vi "UHR-Fleezers Control (host) - 12.8.vi"() -> ()   [LabVIEW 2012] (continued)
  T33 = cluster{"Left":i32, "Top":i32, "Width":u32, "Height":u32}
  T34 = cluster{cluster{"Left":i32, "Top":i32, "Width":u32, "Height":u32}}[]
  T35 = enum32{"setting", "request", "request control", "info", "statistics", "system settings", "I/O sub system", "HRT control", "camera descriptions", "device specific data", "event sub system settings", "event sub system results", "image memory manager"}
  T36 = typedef "IMAQ AVI2 Refnum.ctl" = refnum<k20>
  T37 = typedef "imagedata.ctl" = cluster{"image type":i32, "image depth":i32, "image":u8[], "mask":u8[], "colors":u32[], "Rectangle":cluster{"left":i16, "top":i16, "right":i16, "bottom":i16}}
  T38 = enum32{"Normal Display", "Dual Display (APD)", "FFT", "High Res Display"}
  T39 = cluster{"Origin Pixel":cluster{"X":sgl, "Y":sgl}, "Angle Relative to Horizontal (deg)":sgl, "Axis Reference":u32}
  T40 = typedef "Simple Grid Descriptor" = cluster{"X Step":sgl, "Y Step":sgl, "Unit":T41}
  T41 = typedef "Image Unit" = enum32{"Undefined", "Angström", "Micrometer", "Millimeter", "Centimeter", "Meter", "Kilometer", "Microinch", "Inch", "Feet", "Nautical miles", "Standard miles", "Steps"}
  T42 = cluster{"averaging mode":u16, "weighting mode":u16, "number of averages":u32}
  T43 = cluster{"dB On (F)":bool, "unwrap phase (F)":bool, "convert to degree (F)":bool}
  T44 = cluster{string, string, string, string, string, string, string, string}
  T45 = cluster{string, string, string, string, string, string, string, string, string, string, string, string}
  T46 = cluster{string, string, string, string, string, string, string, string, string, string, string, string, string}
  T47 = cluster{string, string, string, string, string, string, string, string, string, string, string, string, string, string}
  T48 = cluster{"BD 1 Frequency 1 (MHz)":dbl, "BD 1 Frequency 2 (MHz)":dbl}
  T49 = cluster{"f0":dbl, "df":dbl, "magnitude":dbl[]}[][]
  T50 = cluster{"Comment (data description)":string, "Channel 1 Buffer":string, "Channel 2 Buffer":string, "Channel 3 Buffer":string, "Title":string, "DNA Construct":string, "Bead diameter":dbl, "Name":string}
diagram:
  w18 = u16 10 items=["1.0"=10, "1.5"=15, "2.0"=20] ("stop bits (10: 1 bit)")
  w34 = u16 20 items=["1.0"=10, "1.5"=15, "2.0"=20] ("stop bits (10: 1 bit)")
  w37 = u16 20 items=["1.0"=10, "1.5"=15, "2.0"=20] ("stop bits (10: 1 bit)")
  w45 = u16 20 items=["1.0"=10, "1.5"=15, "2.0"=20] ("stop bits (10: 1 bit)")
  w24 = T19 2 items=["Grayscale (U8)", "Grayscale (I16)", "Grayscale (SGL)", "Complex (CSG)", "RGB (U32)", "HSL (U32)", "RGB (U64)", "Grayscale (U16)"] ("Image Type")
  # "Settings to help prevent AOM/D damage"
  # "Initialize the FPGA DAQ card itself"
  # "Reset the DAQ card."
  # "Specify the DAQ card and the FPGA code to run"
  # "Bottom 1 Harvard"
  # "Top 3 Harvard"
  # "Center Harvard"
  # "Bottom 1 Harvard"
  # "Top 3 Harvard"
  # "Center Harvard"
  n1 = case "Trap X limits" shown="\"AOD3Sets\"" "1axis AOM vs 2 axis AOD" {
    tunnel: [T16 {"Minimum"=0.0, "Maximum"=40.0, "Increment"=0.1} ("Min Max Inc") T16 {"Minimum"=0.0, "Maximum"=40.0, "Increment"=0.1} ("Min Max Inc") T16 {"Minimum"=60.0, "Maximum"=90.0, "Increment"=1.0} ("Min Max Inc")] -> w9
    tunnel: [T16 {"Minimum"=0.0, "Maximum"=45.0, "Increment"=1.0} ("Data Entry Limits") T16 {"Minimum"=0.0, "Maximum"=45.0, "Increment"=1.0} ("Data Entry Limits") T16 {"Minimum"=0.0, "Maximum"=50.0, "Increment"=1.0} ("Data Entry Limits")] -> w7
    frame "2axisAOD" {
      w81 = u16 300 ("DIO count 1 (ticks)")
      # "Amp Limits"
      # "Freq Limits"
      n2 = disable-structure shown="Disabled" {
        frame Disabled {
          w87 = 35.0 ("BD 1 Amplitude 1 (%)")
          w88 = 30.0 ("BD 1 Frequency 1 (MHz)")
          n3 = local write "BD 1 Frequency 1 (MHz)"(w88) -> ()
          n4 = local write "BD 1 Frequency 2 (MHz)"(w88) -> ()
          n5 = local write "BD 1 Amplitude 2 (%)"(w87) -> ()
          n6 = local write "BD 1 Amplitude 1 (%)"(w87) -> ()
          n7 = local write "BD 2 Frequency 1 (MHz)"(w88) -> ()
          n8 = local write "BD 2 Amplitude 1 (%)"(w87) -> ()
          n9 = local write "BD 2 Frequency 2 (MHz)"(w88) -> ()
          n10 = local write "BD 2 Amplitude 2 (%)"(w87) -> ()
        }
        frame Enabled {
        }
      }
      n11 = local write "All FB On/Off"(FALSE ("All FB On/Off")) -> ()
      n12 = local write "BD 2 Delay (Ticks)"(u8 108 ("BD 2 Delay (Ticks)")) -> ()
      n13 = local write "Number Interlace Sets"(u8 2 ("Number Interlace Sets")) -> ()
      n14 = local write "DIO count 2 (ticks)"(w81) -> ()
      n15 = local write "DIO count 1 (ticks)"(w81) -> ()
    }
    frame "AOD3Sets" {
      w89 = u16 200 ("DIO count 1 (ticks)")
      # "Amp Limits"
      # "Freq Limits"
      n16 = disable-structure shown="Disabled" {
        frame Disabled {
          w95 = 35.0 ("BD 1 Amplitude 1 (%)")
          w96 = 30.0 ("BD 1 Frequency 1 (MHz)")
          n17 = local write "BD 1 Frequency 1 (MHz)"(w96) -> ()
          n18 = local write "BD 1 Frequency 2 (MHz)"(w96) -> ()
          n19 = local write "BD 1 Amplitude 2 (%)"(w95) -> ()
          n20 = local write "BD 1 Amplitude 1 (%)"(w95) -> ()
          n21 = local write "BD 2 Frequency 1 (MHz)"(w96) -> ()
          n22 = local write "BD 2 Amplitude 1 (%)"(w95) -> ()
          n23 = local write "BD 2 Frequency 2 (MHz)"(w96) -> ()
          n24 = local write "BD 2 Amplitude 2 (%)"(w95) -> ()
        }
        frame Enabled {
        }
      }
      n25 = local write "All FB On/Off"(FALSE ("All FB On/Off")) -> ()
      n26 = local write "BD 2 Delay (Ticks)"(u8 0 ("BD 2 Delay (Ticks)")) -> ()
      n27 = local write "Number Interlace Sets"(u8 3 ("Number Interlace Sets")) -> ()
      n28 = local write "DIO count 2 (ticks)"(w89) -> ()
      n29 = local write "DIO count 1 (ticks)"(w89) -> ()
    }
    frame "1axis", Default {
      # "Amp Lmits"
      # "Freq Limits"
    }
  }
  n30 = xnode "Open FPGA VI Reference"("resource name"=T18 "750kHzDAQ") -> ("FPGA VI Reference Out"=w14:T20, "error out"=w13:errorcluster)  [unwired: 1 in]
  n31 = xnode "Invoke Method"("FPGA VI Reference In"=w14, "error in"=w13) -> ("FPGA VI Reference Out"=w6:T20, "error out"=→"FPGA error out":errorcluster)
  n32 = flat-sequence "Safety limits on RF frequencies and amplitudes (for AOM protection)" {
    tunnel: [w101] -> w1
    tunnel: [w100] -> w3
    tunnel: [w102] -> w4
    tunnel: [w103] -> w2
    tunnel: w9 -> [w101]
    tunnel: w7 -> [w100]
    tunnel: w6 -> [w99]
    tunnel: [w99] -> w5
    frame #0 {
      w103 = T16 {"Minimum"=0.0, "Maximum"=40.0, "Increment"=0.1} ("Min Max Inc")
      w102 = T16 {"Minimum"=0.0, "Maximum"=45.0, "Increment"=1.0} ("Data Entry Limits")
      n33 = property on="BD 2 Frequency 1 (MHz)" class="DigNum (strict)"("Data Range"=w103) -> ()  [unwired: 2 in, 2 out]
      n34 = property on="BD 2 Frequency 3 (MHz)" class="DigNum (strict)"("Data Range"=w103) -> ()  [unwired: 2 in, 2 out]
      n35 = property on="BD 2 Frequency 2 (MHz)" class="DigNum (strict)"("Data Range"=w103) -> ()  [unwired: 2 in, 2 out]
      n36 = property on="BD 1 Frequency 1 (MHz)" class="DigNum (strict)"("Data Range"=w101) -> ()  [unwired: 2 in, 2 out]
      n37 = property on="BD 1 Frequency 2 (MHz)" class="DigNum (strict)"("Data Range"=w101) -> ()  [unwired: 2 in, 2 out]
      n38 = property on="BD 1 Frequency 3 (MHz)" class="DigNum (strict)"("Data Range"=w101) -> ()  [unwired: 2 in, 2 out]
      n39 = property on="BD 2 Amplitude 1 (%)" class="DigNum (strict)"("Data Range"=w102) -> ()  [unwired: 2 in, 2 out]
      n40 = property on="BD 2 Amplitude 2 (%)" class="DigNum (strict)"("Data Range"=w102) -> ()  [unwired: 2 in, 2 out]
      n41 = property on="BD 2 Amplitude 3 (%)" class="DigNum (strict)"("Data Range"=w102) -> ()  [unwired: 2 in, 2 out]
      n42 = property on="BD 1 Amplitude 3 (%)" class="DigNum (strict)"("Data Range"=w100) -> ()  [unwired: 2 in, 2 out]
      n43 = property on="BD 1 Amplitude 2 (%)" class="DigNum (strict)"("Data Range"=w100) -> ()  [unwired: 2 in, 2 out]
      n44 = property on="BD 1 Amplitude 1 (%)" class="DigNum (strict)"("Data Range"=w100) -> ()  [unwired: 2 in, 2 out]
      "X RF Frequency Limits (MHz)" <- w101
      "X RF Amplitude Limits (%)" <- w100
      "Y RF Amplitude Limits (%)" <- w102
      "Y RF Frequency Limits (MHz)" <- w103
    }
  }
  n45 = stacked-sequence "Host initialization sequence - order matters!" {
    tunnel: w5 -> [_ w106 w204 _ w271 w279 w325 w350 w380]
    tunnel: [_ _ _ _ _ _ _ _ w380] -> w11
    tunnel: [_ _ _ _ _ _ _ _ w379] -> w10
    tunnel: w4 -> [_ _ _ _ _ _ w322 _ _]
    tunnel: w3 -> [_ _ _ _ _ _ w321 _ _]
    tunnel: w2 -> [_ _ _ _ _ _ w320 _ _]
    tunnel: w1 -> [_ _ _ _ _ _ w319 _ _]
    frame #0 {
    }
    frame #1 {
      w139 = 10.0 ("y")
      w140 = 32767.0 ("y")
      w124 = 6.0  # clock mult.
      w123 = 49152000.0  # TCXO frequ.
      # "Initialize some FPGA settings"
      n46 = Build Array("DIO count 1 (ticks)", "DIO count 2 (ticks)", "DIO count 3 (ticks)") -> (w174:u16[])
      n47 = local read "AO1"() -> (w145:dbl)
      n48 = local read "AO2"() -> (w146:dbl)
      n49 = local read "Scan Increment (MHz)"() -> (w128:dbl)
      n50 = property on="AI Count (ticks)" class="DigNum (strict)"("Val(Sgnl)"="AI Count (ticks)") -> ()  [unwired: 2 in, 2 out]
      n51 = local read "Continuous MCL Scanning"() -> (w158:bool)
      n52 = local read "Fast Scan Dir"() -> (w159:bool)
      n53 = local read "Number of scans (MCL)"() -> (w157:u64)
      n54 = Multiply(x=w145, y=w140) -> (x*y=w143:dbl)
      n55 = Multiply(x=w146, y=w140) -> (x*y=w141:dbl)
      n56 = Divide(x=40000000.0, y="AI Count (ticks)") -> (x/y=w163:dbl)
      n57 = Divide(x=w143, y=w139) -> (x/y=w144:dbl)
      n58 = Divide(x=w141, y=w139) -> (x/y=w142:dbl)
      n59 = To Word Integer(number=w144) -> (16bit integer=w147:i16)
      n60 = To Word Integer(number=w142) -> (16bit integer=w148:i16)
      n61 = Not(x=w159) -> (.not. x?=w160:bool)
      n62 = local read "Cycles/step (MCL)"() -> (w156:u64)
      n63 = Multiply(x=w128, y=1000.0) -> (x*y=w121:dbl)
      n64 = local read "Scan steps (MCL)"() -> (w155:u64)
      n65 = local write "Trap Pos FIFO Timeout"(u16 0 ("Trap Pos FIFO Timeout")) -> ()
      n66 = local read "Desired Scan Incr (V)"() -> (w153:dbl)
      n67 = local write "AI rate (Hz)"(w163) -> ()
      n68 = Scale By Power Of 2(n=48, x=w121) -> (x*2^n=w120:dbl)
      n69 = Unbundle By Name(cluster{"output high":i16, "output low":i16} {"output high"=3000, "output low"=0} ("FB output range 1")) -> ("output high"=w193:i16, "output low"=w194:i16)
      n70 = Multiply(x=w123, y=w124) -> (x*y=w125:dbl)
      n71 = Divide(x=w120, y=w125) -> (x/y=w126:dbl)
      n72 = local read "Setpoints (V)"() -> (w113:cluster{"Set 1":dbl, "Set 2":dbl})
      n73 = To Quad Integer(1:w126) -> (0:w129:i64)
      n74 = Multiply(x=w153, y=32767.0) -> (x*y=w151:dbl)
      n75 = Divide(x=w163, y="FPGA Ave.") -> (x/y=w162:dbl)
      n76 = local read "Trap Intensity PID Gains"() -> (w118:T9)
      n77 = local read "Next trap write delay (ticks)"() -> (w197:u8)
      n78 = local read "XY phase ext loop method"() -> (w198:bool)
      n79 = local read "Amp switch delay 2"() -> (w199:u8)
      n80 = local read "BD 2 Delay (Ticks) 2"() -> (w200:u8)
      n81 = local read "BD 1 Delay (ticks) 2"() -> (w201:u8)
      n82 = local write "Ave. Rate (Hz)"(w162) -> ()
      n83 = Reciprocal(x=w162) -> (1/x=w161:dbl)
      n84 = local read "Number Interlace Sets"() -> (w181:u8)
      n85 = Split 1D Array(array=w174, index=w181) -> (first subarray=w172:u16[])  [unwired: 1 out]
      n86 = Add Array Elements(numeric array=w172) -> (sum=w173:u16)
      n87 = local write "Ave. Period (s)"(w161) -> ()
      n88 = local read "# Samples/channel"() -> (w136:u32)
      n89 = local read "Number of F/B Scans (AOD)"() -> (w135:u16)
      n90 = local read "Not-Interlacing Set"() -> (w182:enum32{"Set 1", "Set 2", "Set 3"})
      n91 = To Unsigned Byte Integer(number=w182) -> (unsigned 8bit integer=w176:u8)
      n92 = Index Array(array=w174, index=w176) -> (element=w175:u16)
      n93 = local read "Feedback On/Off"() -> (w110:cluster{"Set 1":bool, "Set 2":bool})
      n94 = local read "BD 2 Delay (Ticks)"() -> (w196:u8)
      n95 = local read "BD 1 Delay (ticks)"() -> (w195:u8)
      n96 = local read "Scan steps (AOD)"() -> (w130:u64)
      n97 = local read "All FB On/Off"() -> (w109:bool)
      n98 = local read "Cycles/step (AOD)"() -> (w131:u64)
      n99 = Divide(x=w151, y=10.0) -> (x/y=w152:dbl)
      n100 = Multiply(x=w130, y=w131) -> (x*y=w132:u64)
      n101 = Unbundle By Name(w118) -> ("proportional gain (Kc)"=w189:i16, "integral gain (Kc*Ts/Ti)"=w190:i16, "derivative gain (Kc*Td/Ts)"=w191:i16)
      n102 = Multiply(x=3276.7, y=w113) -> (x*y=w114:cluster{"Set 1":dbl, "Set 2":dbl})
      n103 = To Word Integer(number=w152) -> (16bit integer=w154:i16)
      n104 = Multiply(x=w132, y=u64 2) -> (x*y=w134:u64)
      n105 = To Word Integer(number=w114) -> (16bit integer=w115:cluster{"Set 1":i16, "Set 2":i16})
      n106 = Multiply(x=w134, y=w135) -> (x*y=w137:u64)
      n107 = local read "Sets to FIFO (Traps)"() -> (w185:T15)
      n108 = Divide(x=w137, y=w136) -> (x/y=w138:dbl)
      n109 = Unbundle By Name(w115) -> ("Set 1"=w116:i16, "Set 2"=w117:i16)
      n110 = local read "2D or 1D Scan"() -> (w171:bool)
      n111 = local write "Data points/scans"(w137) -> ()
      n112 = local read "Scan BD"() -> (w119:bool)
      n113 = And(x=w110, y=w109) -> (x .and. y?=w111:cluster{"Set 1":bool, "Set 2":bool})
      n114 = local write "Data points/scan (f/b)"(w134) -> ()
      n115 = local read "N Acq Sets (Traps + Fl.)"() -> (w167:i16)
      n116 = local write "N sets should be saved"(w138) -> ()
      n117 = local read "FPGA error out"() -> (w105:errorcluster)
      n118 = Unbundle By Name(w111) -> ("Set 1"=w107:bool, "Set 2"=w108:bool)
      n119 = local read "Interlace"() -> (w180:bool)
      n120 = Select(t=w173, s=w180, f=w175) -> (s? t:f=w183:u16)
      n121 = local write "Update Count (MCL)"(w183) -> ()
      n122 = local write "Total Counts (ticks)"(w183) -> ()
      n123 = Unbundle By Name(w185) -> ("Set 1"=w186:bool, "Set 2"=w187:bool, "Set 3"=w188:bool)
      n124 = property on="2D or 1D Scan" class="Bool (strict)"("Val(Sgnl)"=w171) -> ()  [unwired: 2 in, 2 out]
      n125 = xnode "Read/Write Control"("FPGA VI Reference In"=w106, "error in"=w105, "ai count"="AI Count (ticks)", "Interlace ON/OFF"=w180, "Number Interlace Cycles"=w181, "Set 1"=w186, "Set 2"=w187, "Set 3"=w188, "FB On/Off Set 1"=w107, "FB On/Off Set 2"=w108, "Interlace Off Parameters"=w182, "FB Setpoint Set 1"=w116, "FB Setpoint Set 2"=w117, "P1"=w189, "I1"=w190, "D1"=w191, "FB1 output high"=w193, "FB1 output low"=w194, "Cycles per step"=w131, "Scan BD"=w119, "Number of scans"=w135, "Scan steps"=w130, "Scan freq.  increment"=w129, "AO1"=w147, "AO2"=w148, "Scan freq.  increment (MCL)"=w154, "Scan steps (MCL)"=w155, "Cycles per step (MCL)"=w156, "Number of scans (MCL)"=w157, "MCL count"=w183, "Cont. Scan (MCL)"=w158, "MCL Scan Axis"=w160, "1D or 2D Scan?"=w171, "N of AI1 Int Acq Sets"=w167, "Amp switch delay"="Amp switch delay", "Swap F1 and F2"="Swap F1 and F2", "APD to FIFO"=FALSE, "DIO count 1 (ticks)"="DIO count 1 (ticks)", "DIO count 2 (ticks)"="DIO count 2 (ticks)", "DIO count 3 (ticks)"="DIO count 3 (ticks)", "BD 1 Delay (ticks)"=w195, "BD 2 Delay (Ticks)"=w196, "Next trap write delay (ticks)"=w197, "XY phase ext loop method"=w198, "Amp switch delay 2"=w199, "BD 2 Delay (Ticks) 2"=w200, "BD 1 Delay (ticks) 2"=w201) -> ("error out"=w104:errorcluster)  [unwired: 1 in, 1 out]
      n126 = local write "FPGA error out"(w104) -> ()
    }
    frame #2 {
      # "Initialize some more FPGA settings"
      n127 = local read "Laser interlacing mode"() -> (w205:enum32{"Laser ON", "Laser OFF", "Interlace"})
      n128 = local read "Green Laser ON"() -> (w206:bool)
      n129 = local read "Trap Pos. FB Range"() -> (w228:T12)
      n130 = local read "Trap Pos. FB Gains"() -> (w229:T11)
      n131 = Multiply(x="Green Intensity % (FB OFF)", y=655.35) -> (x*y=w211:dbl)
      n132 = local read "Invert laser interlacing"() -> (w248:bool)
      n133 = local read "Trap Pos. AI1 X Pre-scale"() -> (w222:u16)
      n134 = Multiply(x="Green FB Setpoint (mV)", y=3.2767) -> (x*y=w214:dbl)
      n135 = local read "Trap Pos FB Int Count"() -> (w224:u16)
      n136 = local read "Differential FB?"() -> (w227:bool)
      n137 = local read "Neg. TTrig FPGA"() -> (w225:bool)
      n138 = Multiply(x="Red FB Setpoint (mV)", y=3.2767) -> (x*y=w240:dbl)
      n139 = To Unsigned Word Integer(number=w211) -> (unsigned 16bit integer=w213:u16)
      n140 = Multiply(x="Red Intensity % (FB OFF)", y=655.35) -> (x*y=w244:dbl)
      n141 = To Word Integer(number=w214) -> (16bit integer=w216:i16)
      n142 = Unbundle By Name("Green FB Gains") -> ("proportional gain (Kc)"=w237:i16, "integral gain (Kc*Ts/Ti)"=w238:i16, "derivative gain (Kc*Td/Ts)"=w239:i16)
      n143 = Unbundle By Name("Red FB Gains") -> ("proportional gain (Kc)"=w251:i16, "integral gain (Kc*Ts/Ti)"=w252:i16, "derivative gain (Kc*Td/Ts)"=w253:i16)
      n144 = case shown="False" w206 {
        tunnel: w205 -> [_ w256]
        tunnel: [enum32{"Laser ON", "Laser OFF", "Interlace"}."Laser OFF" ("Green laser mode") w256] -> w249
        frame False {
        }
        frame True {
        }
      }
      n145 = To Word Integer(number=w240) -> (16bit integer=w243:i16)
      n146 = Unbundle By Name(w229) -> ("proportional gain (Kc)"=w233:fxp<+/-,16,8>, "integral gain (Kc*Ts/Ti)"=w234:fxp<+/-,16,8>, "derivative gain (Kc*Td/Ts)"=w235:fxp<+/-,16,8>)
      n147 = To Unsigned Word Integer(number=w244) -> (unsigned 16bit integer=w247:u16)
      n148 = Unbundle By Name(w228) -> ("output high"=w230:fxp<+/-,16,1>, "output low"=w232:fxp<+/-,16,1>)
      n149 = local read "Trap Pos FB Monitor\nT1 or T2"() -> (w217:bool)
      n150 = local read "Trap Pos FB Negate Action"() -> (w218:bool)
      n151 = local read "Trap Pos. FB Offset Factor"() -> (w219:i64)
      n152 = local read "Trap Pos. FB Mult Factor"() -> (w220:i64)
      n153 = local read "FPGA error out"() -> (w202:errorcluster)
      n154 = xnode "Read/Write Control"("FPGA VI Reference In"=w204, "error in"=w202, "Invert GI 2"=w248, "Operating Mode 2"=w249, "P3"=w237, "I3"=w238, "D3"=w239, "Green FB Setpoint"=w216, "Green FB On/Off"="Green FB On/Off", "Current Out"=w213, "Green int current ON count adj"="Green int current ON count adj", "Operating Mode"=w249, "Invert GI"=w248, "Trap Pos FB Monitor T1 or T2"=w217, "Trap Pos FB Negate Action"=w218, "Trap Pos. FB Offset Factor"=w219, "Trap Pos. FB Mult Factor"=w220, "Force feedback"=FALSE, "AI1 X Scale"=w222, "Trap Pos to FIFO"=TRUE, "Trap Pos FB Int Count"=w224, "TTrig Negate Pos"=w225, "FB Trig Integrate"="FB Trig Integrate", "Diff FB Measurement?"=w227, "Negate Diff?"="Negate Diff?", "P2"=w233, "I2"=w234, "D2"=w235, "FB2 output high"=w230, "FB2 output low"=w232, "Red FB Setpoint"=w243, "RI Current Out"=w247, "Red Laser Operating Mode"=w249, "RI Operating Mode 2"=w249, "Invert RI 2"=w248, "Invert RI"=w248, "P4"=w251, "I4"=w252, "D4"=w253, "Red FB On/Off"="Red FB On/Off") -> ("error out"=w203:errorcluster)  [unwired: 1 out]
      n155 = local write "FPGA error out"(w203) -> ()
    }
    frame #3 {
      # "Initialize more settings. Should stop using event loops to initialize."
      # "What are these?"
      n156 = stacked-sequence {
        frame #0 {
          w259 = T21."empty" ("mode")
          # "Clear external fluorescence triggering FIFO"
          # "APD loop counts"
          # "Fluorescence loop counts (rates)"
          n157 = local read "APD Integration Time (s)"() -> (w261:dbl)
          n158 = local read "Interlace ON count"() -> (w262:u16)
          n159 = call "Smart Buffer (DBL) 1.vi"("mode"=w259) -> ()  [unwired: 5 in, 6 out]
          n160 = call "Smart Buffer (DBL) 2.vi"("mode"=w259) -> ()  [unwired: 5 in, 6 out]
          n161 = property on="APD Integration Time (s)" class="DigNum (strict)"("Val(Sgnl)"=w261) -> ()  [unwired: 2 in, 2 out]
          n162 = property on="Interlace ON count" class="DigNum (strict)"("Val(Sgnl)"=w262) -> ()  [unwired: 2 in, 2 out]
          "Number of APDs" <- 3.0 ("Number of APDs")
        }
        frame #1 {
          # "Number of APDs affects\nAPD DMA transfer"
          # "General settings for all lasers:"
          # "And includes all laser\nON/OFF settings"
          # "Fluorescent lasers settings:"
          # "Blue laser settings:"
          n163 = local read "Laser interlacing mode"() -> (w264:enum32{"Laser ON", "Laser OFF", "Interlace"})
          n164 = local read "Invert laser interlacing"() -> (w263:bool)
          n165 = local read "Blue FB On/Off"() -> (w265:bool)
          n166 = property on="Blue FB On/Off" class="Bool (strict)"("Val(Sgnl)"=w265) -> ()  [unwired: 2 in, 2 out]
          n167 = property on="Invert laser interlacing" class="Bool (strict)"("Val(Sgnl)"=w263) -> ()  [unwired: 2 in, 2 out]
          n168 = property on="Laser interlacing mode" class="RadioBtnsControl (strict)"("Val(Sgnl)"=w264) -> ()  [unwired: 2 in, 2 out]
        }
        frame #2 {
          w266 = path "C:/Home/wheeler/Comstock-LabView-Link.udl" ("connection information")
          # "Initialize the database connection"
          n169 = call-poly <vilib>:"DB Tools Open Connection.vi"("connection information"=w266) -> ("connection reference"=w267:T17)  [unwired: 7 in, 1 out]
          "connection reference" <- w267
          n170 = local write "connection reference"(w267) -> ()
          n171 = local write "Database link"(w266) -> ()
        }
        frame #3 {
          n172 = Wait (ms)(milliseconds to wait=u32 5000) -> ()  [unwired: 1 out]
        }
      }
      n173 = local write "Offset (nm)"(0.0 ("Offset (nm)")) -> ()
      n174 = local write "Bead Mean (nm)"(0.0 ("Bead Mean (nm)")) -> ()
    }
    frame #4 {
      # "Set FIFO size and run FPGA"
      n175 = local read "FPGA error out"() -> (w270:errorcluster)
      n176 = xnode "Invoke Method"("FPGA VI Reference In"=w271, "error in"=w270, "Requested Depth"="Trap AI FIFO Depth") -> ("FPGA VI Reference Out"=w275:T20, "error out"=w276:errorcluster)  [unwired: 1 out]
      n177 = xnode "Invoke Method"("FPGA VI Reference In"=w275, "error in"=w276, "Requested Depth"="Trap Position FIFO Depth") -> ("FPGA VI Reference Out"=w273:T20, "error out"=w272:errorcluster)  [unwired: 1 out]
      n178 = xnode "Invoke Method"("FPGA VI Reference In"=w273, "error in"=w272) -> ("error out"=w269:errorcluster)  [unwired: 1 in, 1 out]
      n179 = local write "FPGA error out"(w269) -> ()
    }
    frame #5 {
      # "Adjust FPGA timing loop phases"
      n180 = flat-sequence "Initial FPGA Loop Relative Phase Adjustment" {
        tunnel: "Initial Phase Adjustment (AI1)" -> [w310]
        tunnel: "Initial Phase Adjustment (GI)" -> [w309]
        tunnel: "Initial Phase Adj. (MCL)" -> [w308]
        tunnel: [w311] -> w295
        tunnel: [w307] -> w294
        tunnel: "Initial Phase Adjustment (APD Acq)" -> [w306]
        tunnel: "Initial Phase Adjustment (APD 1 Gate)" -> [w305]
        tunnel: "Initial Phase Adjustment (Green FB)" -> [w304]
        tunnel: "Initial Phase Adjustment (GI) 2" -> [w303]
        tunnel: "Initial Phase Adjustment (APD 2 Gate)" -> [w302]
        tunnel: "Initial Phase Adjustment (RI)" -> [w301]
        tunnel: "Initial Phase Adjustment (BI DO)" -> [w300]
        tunnel: "Initial Phase Adjustment (BI AO)" -> [w299]
        tunnel: "Initial Phase Adjustment (APD 3 Gate)" -> [w298]
        tunnel: w279 -> [w297]
        tunnel: w295 -> [w313]
        tunnel: [w314] -> w293
        tunnel: w294 -> [w314]
        tunnel: [w313] -> w292
        tunnel: w293 -> [w318]
        tunnel: w292 -> [w317]
        tunnel: [w315] -> w278
        frame #0 {
          n181 = local read "FPGA error out"() -> (w296:errorcluster)
          n182 = xnode "Read/Write Control"("FPGA VI Reference In"=w297, "error in"=w296, "Phase count adjustment"=w310, "Phase count adjustment (GI)"=w309, "Phase count adjustment (MCL)"=w308, "Phase Count Adjustment (APD Acq)"=w306, "Phase count adjustment (APD 1 Gate)"=w305, "Phase count adjustment (APD 2 Gate)"=w302, "Phase count adjustment (Green FB)"=w304, "Phase count adjustment (GI) 2"=w303, "Phase count adjustment (RI)"=w301, "Phase count adjustment (BI AO)"=w299, "Phase count adjustment (BI D)"=w300, "Phase count adjustment (APD 3 Gate)"=w298) -> ("FPGA VI Reference Out"=w307:T20, "error out"=w311:errorcluster)
        }
        frame #1 {
          n183 = Wait (ms)(milliseconds to wait=u32 100) -> ()  [unwired: 1 out]
        }
        frame #2 {
          w316 = TRUE
          n184 = xnode "Read/Write Control"("FPGA VI Reference In"=w318, "error in"=w317, "+ phase"=w316, "+ phase (GI)"=w316, "+ phase (MCL)"=w316, "+ phase (APD Acq)"=w316, "+ phase (APD 1 Gate)"=w316, "+ phase (APD 2 Gate)"=w316, "+ phase (Green FB)"=w316, "+ phase (GI) 2"=w316, "+ phase (RI)"=w316, "+ phase (BI AO)"=w316, "+ phase (BI D)"=w316, "+ phase (APD 3 Gate)"=w316) -> ("error out"=w315:errorcluster)  [unwired: 1 out]
        }
      }
      n185 = local write "FPGA error out"(w278) -> ()
    }
    frame #6 {
      # "Initialize trap RF synth board and set initial frequencies and amplitudes"
      n186 = local read "FPGA error out"() -> (w324:errorcluster)
      n187 = call "Initialize RF boards - interlace 3.vi"("error in"=w324, "FPGA VI Reference In"=w325) -> ("error out"=w326:errorcluster, "FPGA VI Reference Out"=w347:T20)
      n188 = call "set RF board frequency - interlace.vi"("Board 2 Frequency Limits"=w320, "Board 1 Frequency Limits"=w319, "error in"=w326, "FPGA VI Reference In"=w347, "Board 2 Frequency 3 (MHz)"="BD 2 Frequency 3 (MHz)", "Board 1 Frequency 3 (MHz)"="BD 1 Frequency 3 (MHz)", "Board 2 Frequency 2 (MHz)"="BD 2 Frequency 2 (MHz)", "Board 2 Frequency 1 (MHz)"="BD 2 Frequency 1 (MHz)", "Board 1 Frequency 2 (MHz)"="BD 1 Frequency 2 (MHz)", "Board 1 Frequency 1  (MHz)"="BD 1 Frequency 1 (MHz)") -> ("error out"=w330:errorcluster, "FPGA VI Reference Out"=w329:T20)
      n189 = call "set RF board amplitude - interlace.vi"("Board 2 Amplitude Limits"=w322, "Board 1 Amplitude Limits"=w321, "error in"=w330, "FPGA VI Reference In"=w329, "Board 2 Amplitude 3 (%)"="BD 2 Amplitude 3 (%)", "Board 1 Amplitude 3 (%)"="BD 1 Amplitude 3 (%)", "Board 2 Amplitude 2 (%)"="BD 2 Amplitude 2 (%)", "Board 2 Amplitude 1 (%)"="BD 2 Amplitude 1 (%)", "Board 1 Amplitude 2 (%)"="BD 1 Amplitude 2 (%)", "Board 1 Amplitude 1 (%)"="BD 1 Amplitude 1 (%)") -> ("error out"=w323:errorcluster)  [unwired: 1 out]
      n190 = Subtract(x="BD 1 Frequency 1 (MHz)", y="BD 1 Frequency 2 (MHz)") -> (x-y=w337:dbl)
      n191 = Subtract(x="BD 2 Frequency 1 (MHz)", y="BD 2 Frequency 2 (MHz)") -> (x-y=w338:dbl)
      n192 = local write "FPGA error out"(w323) -> ()
      n193 = Square(x=w338) -> (x^2=w340:dbl)
      n194 = Square(x=w337) -> (x^2=w339:dbl)
      n195 = Add(x=w339, y=w340) -> (x+y=w341:dbl)
      n196 = Square Root(x=w341) -> (sqrt(x)=w342:dbl)
      n197 = local write "Trap Delta (MHz)"(w342) -> ()
    }
    frame #7 {
      n198 = local read "FPGA error out"() -> (w349:errorcluster)
      n199 = flat-sequence {
        tunnel: [w364] -> w354
        tunnel: [w363] -> w353
        tunnel: w350 -> [w356]
        tunnel: w349 -> [w355]
        tunnel: [w368] -> w352
        tunnel: w354 -> [w368]
        tunnel: [w367] -> w351
        tunnel: w353 -> [w367]
        tunnel: w352 -> [w376]
        tunnel: w351 -> [w375]
        tunnel: [w370] -> w348
        frame #0 {
          w357 = FALSE ("Retract Pump 3")
          n200 = local read "Trap 1 (ON/OFF)"() -> (w358:bool)
          n201 = xnode "Read/Write Control"("FPGA VI Reference In"=w356, "error in"=w355, "Direct RF Box  Communication"=FALSE) -> ("FPGA VI Reference Out"=w364:T20, "error out"=w363:errorcluster)
          n202 = local write "Saving..."(FALSE ("Saving Data")) -> ()
          n203 = local write "Stop All"(FALSE ("Stop All")) -> ()
          n204 = local write "Retract Pump 1"(w357) -> ()
          n205 = local write "Retract Pump 3"(w357) -> ()
          n206 = local write "Index"(1.0 ("Index")) -> ()
          n207 = property on="Trap 1 ON" class="Bool (strict)"("Value"=w358) -> ()  [unwired: 2 in, 2 out]
          "Manipulating Trap" <- FALSE ("Manipulating Trap")
        }
        frame #1 {
          n208 = local read "Trap 2 (ON/OFF)"() -> (w366:bool)
          n209 = Wait (ms)(milliseconds to wait=u32 10) -> ()  [unwired: 1 out]
          n210 = property on="Trap 2 ON" class="Bool (strict)"("Val(Sgnl)"=w366) -> ()  [unwired: 2 in, 2 out]
        }
        frame #2 {
          n211 = local read "Scan Range (nm)"() -> (w371:dbl)
          n212 = xnode "Read/Write Control"("FPGA VI Reference In"=w376, "error in"=w375, "FPGA Controls  RF Box"=TRUE ("Direct RF Box  Communication")) -> ("error out"=w370:errorcluster)  [unwired: 1 out]
          n213 = call "Update messages.vi"("Message to add"="UHR-Fleezers ready.", "Old message string"="") -> ("New message string"=w374:string)
          n214 = local write "Messages"(w374) -> ()
          n215 = property on="Scan Range (nm)" class="DigNum (strict)"("Val(Sgnl)"=w371) -> ()  [unwired: 2 in, 2 out]
        }
      }
      n216 = local write "FPGA error out"(w348) -> ()
    }
    frame #8 {
      # "Wait 5 s for all the event loops still being executed to finish."
      n217 = Wait (ms)(milliseconds to wait=u32 5000) -> ()  [unwired: 1 out]
      n218 = local read "FPGA error out"() -> (w379:errorcluster)
    }
  }
  n219 = call-poly "VISA Configure Serial Port"("VISA resource name"="VISA resource name", "baud rate (9600)"=u32 115200, "stop bits (10: 1 bit)"=w18) -> ("VISA resource name out"=w17:refnum<visa-resource-name>, "error out"=w16:errorcluster)  [unwired: 4 in, 7 out]
  n220 = call-poly "VISA Configure Serial Port"("VISA resource name"="Bottom  1 Harvard Syringe Pump Serial Port", "baud rate (9600)"=u32 115200, "stop bits (10: 1 bit)"=w34) -> ("VISA resource name out"=w30:refnum<visa-resource-name>, "error out"=w29:errorcluster)  [unwired: 4 in, 7 out]
  n221 = call-poly "VISA Configure Serial Port"("VISA resource name"="Top 3 Harvard Syringe Pump Serial Port", "baud rate (9600)"=u32 115200, "stop bits (10: 1 bit)"=w37) -> ("VISA resource name out"=w32:refnum<visa-resource-name>, "error out"=w31:errorcluster)  [unwired: 4 in, 7 out]
  n222 = call-poly "VISA Configure Serial Port"("VISA resource name"="Sample Chamber Stage Serial Port") -> ("VISA resource name out"=w58:refnum<visa-resource-name>, "error out"=w59:errorcluster)  [unwired: 5 in, 8 out]
  "Stage Control Serial Error" <- w59
  n223 = local write "Blue Error Out"(w16) -> ()
  n224 = call-poly "VISA Configure Serial Port"("VISA resource name"="Center Harvard Syringe Pump Serial Port", "baud rate (9600)"=u32 115200, "stop bits (10: 1 bit)"=w45) -> ("VISA resource name out"=w42:refnum<visa-resource-name>, "error out"=w43:errorcluster)  [unwired: 4 in, 7 out]
  n225 = call "IMAQ Create"("Image Name"="APD 1 Image", "Image Type"=w24) -> ("New Image"=w51:T2)  [unwired: 3 in, 1 out]
  n226 = call "IMAQ Create"("Image Name"="APD 2 Image", "Image Type"=w24) -> ("New Image"=w50:T2)  [unwired: 3 in, 1 out]
  n227 = call "IMAQ Create"("Image Name"="APD 3 Image", "Image Type"=w24) -> ("New Image"=w23:T2)  [unwired: 3 in, 1 out]
  n228 = call "IMAQ Create"("Image Name"="Det. X Image", "Image Type"=w24) -> ("New Image"=w49:T2)  [unwired: 3 in, 1 out]
  n229 = call "IMAQ Create"("Image Name"="Det. Y Image", "Image Type"=w24) -> ("New Image"=w48:T2)  [unwired: 3 in, 1 out]
  n230 = Bundle("New Image"=w51, "New Image"=w50, "New Image"=w23, "New Image"=w49, "New Image"=w48) -> (w47:T22)  [unwired: 1 in]
  n231 = node-c288() -> (w54:T23)  [unwired: 4 in]
  n232 = timed-loop "Run Scripts, including: stage motion" {
    tunnel: w59 -> [w389]
    tunnel: w58 -> [w390]
    tunnel: [w390] -> w57
    tunnel: [w389] -> w56
    timing: w54 -> [_]
    timing-out: [_] -> w53
    tunnel: w42 -> [w388]
    tunnel: w43 -> [w387]
    tunnel: w32 -> [w384]
    tunnel: w31 -> [w383]
    tunnel: w30 -> [w385]
    tunnel: w29 -> [w386]
    tunnel: w17 -> [w382]
    tunnel: w5 -> [w381]
    stop <- w391 stop-if-true
    n233 = node-c288() -> ()  [unwired: 1 in, 1 out]
    n234 = event shown="[11] \"-y\", \"+y\": Value Change" {
      selector: _ -> [_ _ _ _ _ _ _ _ _ _ _ _ _ _ _ _ _ _ _ _ _ _ _ _ _ _]
      dyn-events: _ -> [_ _ _ _ _ _ _ _ _ _ _ _ _ _ _ _ _ _ _ _ _ _ _ _ _ _]
      timeout: _ -> [_ _ _ _ _ _ _ _ _ _ _ _ _ _ _ _ _ _ _ _ _ _ _ _ _ _]
      tunnel: ["Set Position" "Move to Position" _ _ _ _ _ _ "Read Harvard" _ _ _ _ _ _ _ _ "Got ADig bead" "Force FB Data\nScript" _ "Got DNA bead" "Take Stepping Data" _ "Take Detection Laser\nImage" _ _] -> _
      tunnel: [_ _ _ _ _ _ _ _ _ _ _ _ _ _ _ _ _ _ _ _ _ _ _ _ _ w1283] -> w391
      tunnel: w389 -> [w409 w417 w430 w460 _ _ _ _ _ w576 w610 w644 w684 w765 w794 w926 w952 _ w988 _ _ _ _ _ _ _]
      tunnel: w390 -> [w410 w418 w431 w461 _ _ _ _ _ w577 w611 w645 w685 w766 w795 w927 w953 _ w989 _ _ _ _ _ _ _]
      tunnel: w388 -> [_ _ _ _ _ _ _ _ w561 _ _ _ _ _ _ _ _ _ _ _ _ _ _ _ _ _]
      tunnel: w387 -> [_ _ _ _ _ _ _ _ w560 _ _ _ _ _ _ _ _ _ _ _ _ _ _ _ _ _]
      tunnel: w386 -> [_ _ _ _ _ _ _ _ _ _ _ _ _ _ _ _ _ _ _ _ _ _ _ _ _ _]
      tunnel: w385 -> [_ _ _ _ _ _ _ _ _ _ _ _ _ _ _ _ _ _ _ _ _ _ _ _ _ _]
      tunnel: w384 -> [_ _ _ _ _ _ _ _ _ _ _ _ _ _ _ _ _ _ _ _ _ _ _ _ _ _]
      tunnel: w383 -> [_ _ _ _ _ _ _ _ _ _ _ _ _ _ _ _ _ _ _ _ _ _ _ _ _ _]
      tunnel: w382 -> [_ _ _ _ w488 w516 w540 w551 _ _ _ _ _ _ _ _ _ _ _ _ _ _ _ _ _ w1282]
      tunnel: w381 -> [_ _ _ _ _ _ _ _ _ _ _ _ _ _ _ _ _ _ _ _ _ _ _ _ w1149 _]
      event "Set Position", "Set Position 2", "Set Position 3", "Set Position 4", "Set Position 5", "Set Position 1": Value Change {
        n235 = event-data() -> ()  [unwired: 1 in, 5 out]
        n236 = Build Array("Set Position 1", "Set Position 2", "Set Position 3", "Set Position 4", "Set Position 5") -> (w408:bool[])
        n237 = Boolean Array To Number(Boolean array=w408) -> (number=w407:u32)
        n238 = Logarithm Base 2(1:w407) -> (0:w399:dbl)
        n239 = call "Read Stage Position.vi"("error in"=w409, "VISA resource name in"=w410) -> ("Current Position"=w414:cluster{dbl, dbl, dbl}, "error out"=w413:errorcluster)  [unwired: 2 out]
        n240 = Decrement(x="Position") -> (x-1=w397:dbl)
        n241 = Greater Or Equal?(x=w399, y=0.0) -> (x >= y?=w400:bool)
        n242 = Cluster To Array(cluster=w414) -> (array=w411:dbl[])
        n243 = local write "Stage Control Serial Error"(w413) -> ()
        n244 = Select(t=w399, s=w400, f=w397) -> (s? t:f=w396:dbl)
        n245 = Increment(x=w396) -> (x+1=w395:dbl)
        n246 = Build Array (concatenate)(w395, w411) -> (w394:dbl[])
        n247 = Replace Array Subset(array="Saved Stage Positions", new element=w394, index (row)=w396) -> (w412:dbl[][])  [unwired: 1 in]
        n248 = local write "Saved Stage Positions"(w412) -> ()
      }
      event "Move to Position": Value Change {
        n249 = event-data() -> ()  [unwired: 1 in, 5 out]
        n250 = flat-sequence {
          tunnel: w418 -> [w422]
          tunnel: w417 -> [w421]
          frame #0 {
            n251 = local read "Saved Stage Positions"() -> (w424:dbl[][])
            n252 = local read "Position"() -> (w423:dbl)
            n253 = local write "Stage Moving"(TRUE ("Stage Moving")) -> ()
            n254 = call "move to saved stage position.vi"("error in"=w421, "Stage VISA resource name in"=w422, "Position"=w423, "Saved Stage Positions"=w424) -> ("error out"=w420:errorcluster)  [unwired: 1 out]
            n255 = local write "Stage Control Serial Error"(w420) -> ()
          }
          frame #1 {
            n256 = call <vilib>:"Beep.vi"() -> ()  [unwired: 3 in, 9 out]
            n257 = local write "Stage Moving"(FALSE ("Stage Moving")) -> ()
          }
        }
      }
      event "Move Cap. 1 (DNA Bottom)": Value Change {
        n258 = event-data() -> ()  [unwired: 1 in, 5 out]
        n259 = local write "Move Cap. 1 (DNA Bottom)"(FALSE ("Move Cap. 1 (DNA Right)")) -> ()
        n260 = flat-sequence {
          tunnel: w430 -> [w433]
          tunnel: w431 -> [w434]
          tunnel: [w434] -> w428
          tunnel: [w433] -> w427
          tunnel: w428 -> [w436]
          tunnel: w427 -> [w435]
          frame #0 {
            n261 = property on="Sample Channel\nFlow" class="Bool (strict)"("Val(Sgnl)"="Cap 1 Samp Flow ON") -> ()  [unwired: 2 in, 2 out]
          }
          frame #1 {
            n262 = local read "Saved Stage Positions"() -> (w446:dbl[][])
            n263 = local write "Stage Moving"(TRUE ("Stage Moving")) -> ()
            n264 = Array Subset(array=w446, index (row)=0 ("index"), length (row)=1 ("length"), index (col)=1 ("index"), length (col)=3 ("length")) -> (w443:dbl[][])
            n265 = Reshape Array(w443, 3 ("dimension size")) -> (w441:dbl[])
            n266 = Array To Cluster(array=w441) -> (cluster=w440:cluster{"[0]":dbl, "[1]":dbl, "[2]":dbl})
            n267 = call "Set Stage Position.vi"("Position"=w440, "error in"=w435, "VISA resource name in"=w436) -> ("error out"=w439:errorcluster)  [unwired: 2 out]
            n268 = local write "Stage Control Serial Error"(w439) -> ()
          }
          frame #2 {
            n269 = local write "Stage Moving"(FALSE ("Stage Moving")) -> ()
            n270 = case shown="True" "Cap 1 Flow ON" {
              frame False {
              }
              frame True {
                n271 = property on="Inject Pump 1" class="Bool (strict)"("Val(Sgnl)"=TRUE ("Value (Signaling)")) -> ()  [unwired: 2 in, 2 out]
              }
            }
            n272 = call <vilib>:"Beep.vi"() -> ()  [unwired: 3 in, 9 out]
          }
          frame #3 {
            n273 = property on="Sample Channel\nFlow" class="Bool (strict)"("Val(Sgnl)"=FALSE ("Value (Signaling)")) -> ()  [unwired: 2 in, 2 out]
            n274 = local read "Cap. 2 BD T1?\n(ADig T1, DNA T2)"() -> (w453:bool)
            n275 = case shown="True" w453 {
              tunnel: "Cap 1 T ON" -> [w455 w456]
              frame False {
                n276 = property on="Trap 1 (ON/OFF)" class="Bool (strict)"("Val(Sgnl)"=w455) -> ()  [unwired: 2 in, 2 out]
              }
              frame True {
                n277 = property on="Trap 2 (ON/OFF)" class="Bool (strict)"("Val(Sgnl)"=w456) -> ()  [unwired: 2 in, 2 out]
              }
            }
            n278 = property on="Got DNA bead" class="Bool"("Key Focus"=TRUE) -> ()  [unwired: 2 in, 2 out]
          }
        }
      }
      event "Move Cap. 2 (ADig Top)": Value Change {
        n279 = event-data() -> ()  [unwired: 1 in, 5 out]
        n280 = local write "Move Cap. 2 (ADig Top)"(FALSE ("Move Cap. 2 (ADig Left)")) -> ()
        n281 = flat-sequence {
          tunnel: w460 -> [w463]
          tunnel: w461 -> [w464]
          tunnel: [w464] -> w458
          tunnel: [w463] -> w457
          tunnel: w458 -> [w467]
          tunnel: w457 -> [w466]
          frame #0 {
            n282 = property on="Sample Channel\nFlow" class="Bool (strict)"("Val(Sgnl)"="Cap 2 Samp Flow ON") -> ()  [unwired: 2 in, 2 out]
          }
          frame #1 {
            w465 = FALSE ("Value (Signaling)")
            n283 = local read "Saved Stage Positions"() -> (w477:dbl[][])
            n284 = local write "Stage Moving"(TRUE ("Stage Moving")) -> ()
            n285 = Array Subset(array=w477, index (row)=1 ("index"), length (row)=1 ("length"), index (col)=1 ("index"), length (col)=3 ("length")) -> (w474:dbl[][])
            n286 = Reshape Array(w474, 3 ("dimension size")) -> (w472:dbl[])
            n287 = property on="Trap 1 (ON/OFF)" class="Bool (strict)"("Val(Sgnl)"=w465) -> ()  [unwired: 2 in, 2 out]
            n288 = property on="Trap 1 (ON/OFF)" class="Bool (strict)"("Val(Sgnl)"=w465) -> ()  [unwired: 2 in, 2 out]
            n289 = Array To Cluster(array=w472) -> (cluster=w471:cluster{"[0]":dbl, "[1]":dbl, "[2]":dbl})
            n290 = call "Set Stage Position.vi"("Position"=w471, "error in"=w466, "VISA resource name in"=w467) -> ("error out"=w470:errorcluster)  [unwired: 2 out]
            n291 = local write "Stage Control Serial Error"(w470) -> ()
          }
          frame #2 {
            n292 = local write "Stage Moving"(FALSE ("Stage Moving")) -> ()
            n293 = call <vilib>:"Beep.vi"() -> ()  [unwired: 3 in, 9 out]
            n294 = case shown="True" "Cap 2 Flow ON" {
              frame False {
              }
              frame True {
                n295 = property on="Inject Pump 3" class="Bool (strict)"("Val(Sgnl)"=TRUE ("Value (Signaling)")) -> ()  [unwired: 2 in, 2 out]
              }
            }
          }
          frame #3 {
            n296 = property on="Sample Channel\nFlow" class="Bool (strict)"("Val(Sgnl)"=FALSE ("Value (Signaling)")) -> ()  [unwired: 2 in, 2 out]
            n297 = case shown="False" "Cap. 2 BD T1?\n(ADig T1, DNA T2)" {
              tunnel: "Cap 2 T ON" -> [w486 w487]
              frame False {
                n298 = property on="Trap 2 (ON/OFF)" class="Bool (strict)"("Val(Sgnl)"=w486) -> ()  [unwired: 2 in, 2 out]
              }
              frame True {
                n299 = property on="Trap 1 (ON/OFF)" class="Bool (strict)"("Val(Sgnl)"=w487) -> ()  [unwired: 2 in, 2 out]
              }
            }
            n300 = property on="Got ADig bead" class="Bool"("Key Focus"=TRUE) -> ()  [unwired: 2 in, 2 out]
          }
        }
      }
      event "Initialize Blue Laser": Value Change {
        n301 = event-data() -> ()  [unwired: 1 in, 5 out]
        n302 = flat-sequence {
          tunnel: w488 -> [w507]
          frame #0 {
            n303 = Concatenate Strings("slmp ", "Blue Laser\nModulation\nPower (mW)") -> (w506:string)
            n304 = call "serial write macro.vi"("String"=w506, "Delay (ms)"="Delay (ms)", "VISA resource name"=w507) -> ("read buffer"=w495:string, "error out"=w496:errorcluster, "VISA resource name out"=w503:refnum<visa-resource-name>)
            n305 = local write "read blue buffer"(w495) -> ()
            n306 = local write "Blue Error Out"(w496) -> ()
            n307 = call "serial write macro.vi"("String"="sdmes 1", "Delay (ms)"="Delay (ms)", "VISA resource name"=w503) -> ("read buffer"=w493:string, "error out"=w494:errorcluster, "VISA resource name out"=w501:refnum<visa-resource-name>)
            n308 = local write "Blue Error Out"(w494) -> ()
            n309 = local write "read blue buffer"(w493) -> ()
            n310 = call "serial write macro.vi"("String"="sames 1", "Delay (ms)"="Delay (ms)", "VISA resource name"=w501) -> ("read buffer"=w490:string, "error out"=w492:errorcluster, "VISA resource name out"=w498:refnum<visa-resource-name>)
            n311 = local write "read blue buffer"(w490) -> ()
            n312 = local write "Blue Error Out"(w492) -> ()
            n313 = call "serial write macro.vi"("String"="l1", "Delay (ms)"="Delay (ms)", "VISA resource name"=w498) -> ("read buffer"=w489:string, "error out"=w491:errorcluster)  [unwired: 1 out]
            n314 = local write "read blue buffer"(w489) -> ()
            n315 = local write "Blue Error Out"(w491) -> ()
          }
          frame #1 {
            n316 = local write "Initialize Blue Laser"(FALSE ("Initialize")) -> ()
          }
        }
      }
      event "Blue Laser Modluation Mode": Value Change {
        # "Changes the type of modulation for the blue laser"
        n317 = event-data() -> ()  [unwired: 1 in, 5 out]
        n318 = case shown="\"Constant Power\"" "Blue Laser Modluation Mode" {
          tunnel: ["sdmes 1" w525 "sdmes 1" "sdmes 0"] -> w510
          tunnel: ["sames 1" "cp" "sames 0" "sames 1"] -> w509
          frame "Digital + Analog", Default {
          }
          frame "Constant Power" {
            n319 = local read "Blue Laser\nModulation\nPower (mW)"() -> (w528:string)
            n320 = Decimal String To Number(string=w528) -> (number=w524:i32)  [unwired: 2 in, 1 out]
            n321 = Divide(x=w524, y=1000) -> (x/y=w522:dbl)
            n322 = Number To Fractional String(number=w522) -> (F-format string=w523:string)  [unwired: 3 in]
            n323 = Concatenate Strings("p ", w523) -> (w525:string)
          }
          frame "Digital Only" {
          }
          frame "Analog Only" {
          }
        }
        n324 = local read "Delay (ms)"() -> (w519:i32)
        n325 = call "serial write macro.vi"("String"=w510, "Delay (ms)"=w519, "VISA resource name"=w516) -> ("read buffer"=w517:string, "error out"=w518:errorcluster, "VISA resource name out"=w511:refnum<visa-resource-name>)
        n326 = local write "read blue buffer"(w517) -> ()
        n327 = local write "Blue Error Out"(w518) -> ()
        n328 = local read "Delay (ms)"() -> (w514:i32)
        n329 = call "serial write macro.vi"("String"=w509, "Delay (ms)"=w514, "VISA resource name"=w511) -> ("read buffer"=w512:string, "error out"=w513:errorcluster)  [unwired: 1 out]
        n330 = local write "Blue Error Out"(w513) -> ()
        n331 = local write "read blue buffer"(w512) -> ()
      }
      event "Blue Laser\nModulation\nPower (mW)": Value Change {
        n332 = event-data() -> ()  [unwired: 1 in, 5 out]
        n333 = local read "Blue Laser\nModulation\nPower (mW)"() -> (w535:string)
        n334 = local read "Blue Laser Modluation Mode"() -> (w536:string)
        n335 = case shown="\"Constant Power\"" w536 {
          tunnel: w535 -> [w542 w549]
          tunnel: [w541 w548] -> w534
          frame "Constant Power" {
            # "Different command to change constant power instead of modulation power"
            n336 = Decimal String To Number(string=w542) -> (offset past number=w547:i32)  [unwired: 2 in, 1 out]
            n337 = Divide(x=w547, y=1000) -> (x/y=w545:dbl)
            n338 = Number To Fractional String(number=w545) -> (F-format string=w543:string)  [unwired: 3 in]
            n339 = Concatenate Strings("p ", w543) -> (w541:string)
          }
          frame Default {
            n340 = Concatenate Strings("slmp ", w549) -> (w548:string)
          }
        }
        n341 = local read "Delay (ms)"() -> (w539:i32)
        n342 = call "serial write macro.vi"("String"=w534, "Delay (ms)"=w539, "VISA resource name"=w540) -> ("read buffer"=w538:string, "error out"=w537:errorcluster)  [unwired: 1 out]
        n343 = local write "Blue Error Out"(w537) -> ()
        n344 = local write "read blue buffer"(w538) -> ()
      }
      event "Send string\nto Blue Laser": Value Change {
        n345 = event-data() -> ()  [unwired: 1 in, 5 out]
        n346 = flat-sequence {
          tunnel: w551 -> [w556]
          frame #0 {
            n347 = local read "Delay (ms)"() -> (w553:i32)
            n348 = call "serial write macro.vi"("String"="command string", "Delay (ms)"=w553, "VISA resource name"=w556) -> ("read buffer"=w554:string, "error out"=→"Blue Error Out":errorcluster)  [unwired: 1 out]
            "read blue buffer" <- w554
            n349 = String Length(string=w554) -> (length=→"length":i32)
            "command string sent" <- "command string"
          }
          frame #1 {
            n350 = local write "Send string\nto Blue Laser"(FALSE ("Send string")) -> ()
          }
        }
      }
      event "Read Harvard": Value Change {
        n351 = event-data() -> ()  [unwired: 1 in, 5 out]
        n352 = Concatenate Strings("write buffer", "\r") -> (w563:string)
        n353 = VISA Write(VISA resource name=w561, write buffer=w563, error in (no error)=w560) -> (VISA resource name out=w572:refnum<visa-resource-name>, error out=w571:errorcluster)  [unwired: 1 out]
        n354 = stacked-sequence {
          tunnel: [w575] -> w570
          tunnel: w572 -> [w575]
          tunnel: w571 -> [w574]
          tunnel: [w574] -> w565
          frame #0 {
            n355 = Wait (ms)(milliseconds to wait=50) -> ()  [unwired: 1 out]
          }
        }
        n356 = property class="Instr"(reference=w570, error in=w565) -> (reference out=w569:refnum<visa-resource-name>, error out=w567:errorcluster, "Serial Settings:Number of Bytes at Serial Port"=w568:u32)
        "Serial Settings:Number of Bytes at Serial Port" <- w568
        n357 = VISA Read(VISA resource name=w569, byte count=w568, error in (no error)=w567) -> (read buffer=w566:string)  [unwired: 3 out]
        "read buffer" <- w566
        n358 = Fract/Exp String To Number(string=w566) -> ()  [unwired: 5 out]
      }
      event "+z", "-z": Value Change {
        n359 = event-data() -> ()  [unwired: 1 in, 5 out]
        n360 = flat-sequence {
          tunnel: w576 -> [w598]
          tunnel: w577 -> [w578]
          frame #0 {
            n361 = call "Read Stage Position.vi"("error in"=w598, "VISA resource name in"=w578) -> ("Current Position"=w583:cluster{dbl, dbl, dbl}, "error out"=w596:errorcluster, "VISA resource name out"=w597:refnum<visa-resource-name>)  [unwired: 1 out]
            n362 = local read "Saved Stage Positions"() -> (w607:dbl[][])
            n363 = Divide(x="z nudge increment (um)", y=1000.0) -> (x/y=w595:dbl)
            n364 = Boolean To (0,1)(Boolean="+z") -> (0, 1=w587:i16)
            n365 = Boolean To (0,1)(Boolean="-z") -> (0, 1=w588:i16)
            n366 = Array Subset(array=w607, index (row)=1 ("index"), length (row)=1 ("length"), index (col)=1 ("index"), length (col)=3 ("length")) -> (w604:dbl[][])
            n367 = Multiply(x=w587, y=w595) -> (x*y=w591:dbl)
            n368 = Multiply(x=w588, y=w595) -> (x*y=w589:dbl)
            n369 = Unbundle(w583) -> (w581:dbl, w580:dbl, w584:dbl)
            n370 = Negate(x=w589) -> (-x=w590:dbl)
            n371 = Reshape Array(w604, 3 ("dimension size")) -> (w602:dbl[])
            n372 = Add(x=w591, y=w590) -> (x+y=w592:dbl)
            n373 = Array To Cluster(array=w602) -> ()  [unwired: 1 out]
            n374 = Add(x=w592, y=w584) -> (x+y=w582:dbl)
            n375 = Bundle(cluster=w583, w581, w580, w582) -> (w579:cluster{dbl, dbl, dbl})
            n376 = call "Set Stage Position.vi"("Position"=w579, "error in"=w596, "VISA resource name in"=w597) -> ("error out"=w601:errorcluster)  [unwired: 2 out]
            n377 = local write "Stage Moving"(TRUE ("Stage Moving")) -> ()
            n378 = local write "Stage Control Serial Error"(w601) -> ()
          }
          frame #1 {
            n379 = local write "Stage Moving"(FALSE ("Stage Moving")) -> ()
          }
        }
      }
      event "-x", "+x": Value Change {
        n380 = event-data() -> ()  [unwired: 1 in, 5 out]
        n381 = flat-sequence {
          tunnel: w610 -> [w635]
          tunnel: w611 -> [w615]
          frame #0 {
            n382 = local read "Saved Stage Positions"() -> (w614:dbl[][])
            n383 = call "Read Stage Position.vi"("error in"=w635, "VISA resource name in"=w615) -> ("Current Position"=w620:cluster{dbl, dbl, dbl}, "error out"=w633:errorcluster, "VISA resource name out"=w634:refnum<visa-resource-name>)  [unwired: 1 out]
            n384 = Divide(x="x nudge increment (um)", y=1000.0) -> (x/y=w632:dbl)
            n385 = Boolean To (0,1)(Boolean="+x") -> (0, 1=w624:i16)
            n386 = Boolean To (0,1)(Boolean="-x") -> (0, 1=w625:i16)
            n387 = Array Subset(array=w614, index (row)=1 ("index"), length (row)=1 ("length"), index (col)=1 ("index"), length (col)=1 ("length")) -> (w639:dbl[][])
            n388 = Multiply(x=w624, y=w632) -> (x*y=w628:dbl)
            n389 = Multiply(x=w625, y=w632) -> (x*y=w626:dbl)
            n390 = Unbundle(w620) -> (w618:dbl, w617:dbl, w621:dbl)
            n391 = Negate(x=w626) -> (-x=w627:dbl)
            n392 = Reshape Array(w639, 1 ("dimension size")) -> (w637:dbl[])
            n393 = Add(x=w628, y=w627) -> (x+y=w629:dbl)
            n394 = Array To Cluster(array=w637) -> ()  [unwired: 1 out]
            n395 = Add(x=w629, y=w621) -> (x+y=w619:dbl)
            n396 = Bundle(cluster=w620, w618, w617, w619) -> (w616:cluster{dbl, dbl, dbl})
            n397 = call "Set Stage Position.vi"("Position"=w616, "error in"=w633, "VISA resource name in"=w634) -> ("error out"=w613:errorcluster)  [unwired: 2 out]
            n398 = local write "Stage Control Serial Error"(w613) -> ()
            n399 = local write "Stage Moving"(TRUE ("Stage Moving")) -> ()
          }
          frame #1 {
            n400 = local write "Stage Moving"(FALSE ("Stage Moving")) -> ()
          }
        }
      }
      event "-y", "+y": Value Change {
        n401 = event-data() -> ()  [unwired: 1 in, 5 out]
        n402 = flat-sequence {
          tunnel: w644 -> [w669]
          tunnel: w645 -> [w649]
          frame #0 {
            n403 = local read "Saved Stage Positions"() -> (w648:dbl[][])
            n404 = call "Read Stage Position.vi"("error in"=w669, "VISA resource name in"=w649) -> ("Current Position"=w654:cluster{dbl, dbl, dbl}, "error out"=w667:errorcluster, "VISA resource name out"=w668:refnum<visa-resource-name>)  [unwired: 1 out]
            n405 = Divide(x="y nudge increment (um)", y=1000.0) -> (x/y=w666:dbl)
            n406 = Boolean To (0,1)(Boolean="+y") -> (0, 1=w658:i16)
            n407 = Boolean To (0,1)(Boolean="-y") -> (0, 1=w659:i16)
            n408 = Array Subset(array=w648, index (row)=1 ("index"), length (row)=1 ("length"), index (col)=1 ("index"), length (col)=2 ("length")) -> (w673:dbl[][])
            n409 = Multiply(x=w658, y=w666) -> (x*y=w662:dbl)
            n410 = Multiply(x=w659, y=w666) -> (x*y=w660:dbl)
            n411 = Unbundle(w654) -> (w652:dbl, w651:dbl, w655:dbl)
            n412 = Negate(x=w660) -> (-x=w661:dbl)
            n413 = Reshape Array(w673, 2 ("dimension size")) -> (w671:dbl[])
            n414 = Add(x=w662, y=w661) -> (x+y=w663:dbl)
            n415 = Array To Cluster(array=w671) -> ()  [unwired: 1 out]
            n416 = Add(x=w663, y=w655) -> (x+y=w653:dbl)
            n417 = Bundle(cluster=w654, w652, w651, w653) -> (w650:cluster{dbl, dbl, dbl})
            n418 = call "Set Stage Position.vi"("Position"=w650, "error in"=w667, "VISA resource name in"=w668) -> ("error out"=w647:errorcluster)  [unwired: 2 out]
            n419 = local write "Stage Control Serial Error"(w647) -> ()
            n420 = local write "Stage Moving"(TRUE ("Stage Moving")) -> ()
          }
          frame #1 {
            n421 = local write "Stage Moving"(FALSE ("Stage Moving")) -> ()
          }
        }
      }
      event "Cal/Data Acq. Spot": Value Change {
        n422 = event-data() -> ()  [unwired: 1 in, 5 out]